vi "FlexMag - 24-03-2023.vi"() -> ()   [LabVIEW 2018] (continued)
        n3540 = local read "CH4_CC_DI"() -> (w5125:bool)
        n3541 = Compound Arithmetic op=OR(w5140, w5139, w5137, w5138) -> (w5141:bool)
        n3542 = case shown="False" w5131 {
          tunnel: [T13."Disabled and Grayed Out" ("Disabled") T13."Enabled" ("Disabled")] -> w5130
          frame False {
          }
          frame True {
          }
        }
        n3543 = case shown="False" w5132 {
          tunnel: [T13."Disabled and Grayed Out" ("Disabled") T13."Enabled" ("Disabled")] -> w5129
          frame False {
          }
          frame True {
          }
        }
        n3544 = case shown="False" w5141 {
          frame False {
            n3545 = local read "CH1_DS_DI"() -> (w5297:bool)
            n3546 = local read "CH2_DS_DI"() -> (w5296:bool)
            n3547 = local read "CH3_DS_DI"() -> (w5294:bool)
            n3548 = local read "CH4_DS_DI"() -> (w5295:bool)
            n3549 = Not(x=w5297) -> (.not. x?=w5298:bool)
            n3550 = Not(x=w5296) -> (.not. x?=w5293:bool)
            n3551 = Not(x=w5294) -> (.not. x?=w5292:bool)
            n3552 = Not(x=w5295) -> (.not. x?=w5291:bool)
            n3553 = property on="ch1_door_open" class="Str"("Visible"=w5298) -> ()  [unwired: 2 in, 2 out]
            n3554 = property on="ch2_door_open" class="Str"("Visible"=w5293) -> ()  [unwired: 2 in, 2 out]
            n3555 = property on="ch3_door_open" class="Str"("Visible"=w5292) -> ()  [unwired: 2 in, 2 out]
            n3556 = property on="ch4_door_open" class="Str"("Visible"=w5291) -> ()  [unwired: 2 in, 2 out]
          }
          frame True {
          }
        }
        n3557 = case shown="False" w5136 {
          tunnel: [T13."Disabled and Grayed Out" ("Disabled") T13."Enabled" ("Disabled")] -> w5135
          frame False {
          }
          frame True {
          }
        }
        n3558 = case shown="False" w5134 {
          tunnel: [T13."Disabled and Grayed Out" ("Disabled") T13."Enabled" ("Disabled")] -> w5133
          frame False {
          }
          frame True {
          }
        }
        n3559 = property on="ch1 cc mbar gui" class="DigNum (strict)"("Visible"=w5128) -> ()  [unwired: 2 in, 2 out]
        n3560 = property on="ch2 cc mbar gui" class="DigNum (strict)"("Visible"=w5127) -> ()  [unwired: 2 in, 2 out]
        n3561 = property on="ch3 cc mbar gui" class="DigNum (strict)"("Visible"=w5126) -> ()  [unwired: 2 in, 2 out]
        n3562 = property on="ch4 cc mbar gui" class="DigNum (strict)"("Visible"=w5125) -> ()  [unwired: 2 in, 2 out]
        n3563 = case shown="True" w5142 {
          frame False {
          }
          frame True {
            n3564 = local write "Warning Message"("Water Flow Problem !\nCheck Connections.." ("Warning Message")) -> ()
          }
        }
        n3565 = local write "Description"(w5164) -> ()
        n3566 = property on="Tp1 set speed gui" class="Bool"("DisabledEnum"=w5135) -> ()  [unwired: 2 in, 2 out]
        n3567 = property on="Tp1 normal speed gui" class="Bool"("DisabledEnum"=w5135) -> ()  [unwired: 2 in, 2 out]
        n3568 = property on="Tp1 low speed gui" class="Bool"("DisabledEnum"=w5135) -> ()  [unwired: 2 in, 2 out]
        n3569 = property on="Tp2 normal speed gui" class="Bool"("DisabledEnum"=w5133) -> ()  [unwired: 2 in, 2 out]
        n3570 = property on="Tp2 set speed gui" class="Bool"("DisabledEnum"=w5133) -> ()  [unwired: 2 in, 2 out]
        n3571 = property on="Tp2 low speed gui" class="Bool"("DisabledEnum"=w5133) -> ()  [unwired: 2 in, 2 out]
        n3572 = property on="Tp3 set speed gui" class="Bool"("DisabledEnum"=w5130) -> ()  [unwired: 2 in, 2 out]
        n3573 = property on="Tp3 normal speed gui" class="Bool"("DisabledEnum"=w5130) -> ()  [unwired: 2 in, 2 out]
        n3574 = property on="Tp3 low speed gui" class="Bool"("DisabledEnum"=w5130) -> ()  [unwired: 2 in, 2 out]
        n3575 = property on="Tp4 set speed gui" class="Bool"("DisabledEnum"=w5129) -> ()  [unwired: 2 in, 2 out]
        n3576 = property on="Tp4 normal speed gui" class="Bool"("DisabledEnum"=w5129) -> ()  [unwired: 2 in, 2 out]
        n3577 = property on="Tp4 low speed gui" class="Bool"("DisabledEnum"=w5129) -> ()  [unwired: 2 in, 2 out]
        n3578 = call <vilib>:"Draw Text at Point.vi"("[user-specified font]"=T12 {"Font Name:"="Bold", "Size"=20, "Strikeout?"=FALSE, "Italic?"=FALSE, "Underline?"=FALSE, "Outline?"=FALSE, "Shadow?"=FALSE, "Bold?"=TRUE}, "desired font(Application)"=T11."User-specified Font", "text"=w5163, "origin"=w5162, "picture"=w5165) -> ("new picture"=→"General View":picture)  [unwired: 5 in, 1 out]
      }
    }
    n3579 = Wait Until Next ms Multiple(millisecond multiple=u32 100) -> ()  [unwired: 1 out]
  }
  n3580 = property on="mp1 timer tab" class="TabCtl (strict)"("Visible"=w86) -> ()  [unwired: 2 in, 2 out]
  n3581 = property on="mp2 timer tab" class="TabCtl (strict)"("Visible"=w86) -> ()  [unwired: 2 in, 2 out]
  n3582 = property on="mp3 timer tab" class="TabCtl (strict)"("Visible"=w86) -> ()  [unwired: 2 in, 2 out]
  n3583 = property on="mp4 timer tab" class="TabCtl (strict)"("Visible"=w86) -> ()  [unwired: 2 in, 2 out]
  n3584 = property on="plvbv1 timer tab" class="TabCtl (strict)"("Visible"=w86) -> ()  [unwired: 2 in, 2 out]
  n3585 = property on="plvbv2 timer tab" class="TabCtl (strict)"("Visible"=w86) -> ()  [unwired: 2 in, 2 out]
  n3586 = property on="plvbv3 timer tab" class="TabCtl (strict)"("Visible"=w86) -> ()  [unwired: 2 in, 2 out]
  n3587 = property on="plvbv4 timer tab" class="TabCtl (strict)"("Visible"=w86) -> ()  [unwired: 2 in, 2 out]
  n3588 = property on="chvbv1 timer tab" class="TabCtl (strict)"("Visible"=w86) -> ()  [unwired: 2 in, 2 out]
  n3589 = property on="chvbv2 timer tab" class="TabCtl (strict)"("Visible"=w86) -> ()  [unwired: 2 in, 2 out]
  n3590 = property on="chvbv3 timer tab" class="TabCtl (strict)"("Visible"=w86) -> ()  [unwired: 2 in, 2 out]
  n3591 = property on="chvbv4 timer tab" class="TabCtl (strict)"("Visible"=w86) -> ()  [unwired: 2 in, 2 out]
  n3592 = property on="bgbv1 timer tab" class="TabCtl (strict)"("Visible"=w86) -> ()  [unwired: 2 in, 2 out]
  n3593 = property on="bgbv2 timer tab" class="TabCtl (strict)"("Visible"=w86) -> ()  [unwired: 2 in, 2 out]
  n3594 = property on="bgbv3 timer tab" class="TabCtl (strict)"("Visible"=w86) -> ()  [unwired: 2 in, 2 out]
  n3595 = property on="bgbv4 timer tab" class="TabCtl (strict)"("Visible"=w86) -> ()  [unwired: 2 in, 2 out]
  n3596 = property on="tpbv1 timer tab" class="TabCtl (strict)"("Visible"=w86) -> ()  [unwired: 2 in, 2 out]
  n3597 = property on="tpbv2 timer tab" class="TabCtl (strict)"("Visible"=w86) -> ()  [unwired: 2 in, 2 out]
  n3598 = property on="tpbv3 timer tab" class="TabCtl (strict)"("Visible"=w86) -> ()  [unwired: 2 in, 2 out]
  n3599 = property on="tpbv4 timer tab" class="TabCtl (strict)"("Visible"=w86) -> ()  [unwired: 2 in, 2 out]
  n3600 = property on="cc1 timer tab" class="TabCtl (strict)"("Visible"=w86) -> ()  [unwired: 2 in, 2 out]
  n3601 = property on="cc2 timer tab" class="TabCtl (strict)"("Visible"=w86) -> ()  [unwired: 2 in, 2 out]
  n3602 = property on="cc3 timer tab" class="TabCtl (strict)"("Visible"=w86) -> ()  [unwired: 2 in, 2 out]
  n3603 = property on="cc4 timer tab" class="TabCtl (strict)"("Visible"=w86) -> ()  [unwired: 2 in, 2 out]
  n3604 = property on="pcgv1 timer tab" class="TabCtl (strict)"("Visible"=w86) -> ()  [unwired: 2 in, 2 out]
  n3605 = property on="pcgv2 timer tab" class="TabCtl (strict)"("Visible"=w86) -> ()  [unwired: 2 in, 2 out]
  n3606 = property on="pcgv3 timer tab" class="TabCtl (strict)"("Visible"=w86) -> ()  [unwired: 2 in, 2 out]
  n3607 = property on="pcgv4 timer tab" class="TabCtl (strict)"("Visible"=w86) -> ()  [unwired: 2 in, 2 out]
  n3608 = property on="tp1 timer tab" class="TabCtl (strict)"("Visible"=w86) -> ()  [unwired: 2 in, 2 out]
  n3609 = property on="tp2 timer tab" class="TabCtl (strict)"("Visible"=w86) -> ()  [unwired: 2 in, 2 out]
  n3610 = property on="tp3 timer tab" class="TabCtl (strict)"("Visible"=w86) -> ()  [unwired: 2 in, 2 out]
  n3611 = property on="tp4 timer tab" class="TabCtl (strict)"("Visible"=w86) -> ()  [unwired: 2 in, 2 out]
  n3612 = property on="sov1 timer tab" class="TabCtl (strict)"("Visible"=w86) -> ()  [unwired: 2 in, 2 out]
  n3613 = property on="sov2 timer tab" class="TabCtl (strict)"("Visible"=w86) -> ()  [unwired: 2 in, 2 out]
  n3614 = property on="sov3 timer tab" class="TabCtl (strict)"("Visible"=w86) -> ()  [unwired: 2 in, 2 out]
  n3615 = property on="sov4 timer tab" class="TabCtl (strict)"("Visible"=w86) -> ()  [unwired: 2 in, 2 out]
  n3616 = property on="ch1 trnsbp left timer tab" class="TabCtl (strict)"("Visible"=w86) -> ()  [unwired: 2 in, 2 out]
  n3617 = property on="ch2 trnsbp right timer tab" class="TabCtl (strict)"("Visible"=w86) -> ()  [unwired: 2 in, 2 out]
  n3618 = property on="ch2 trnsbp left timer tab" class="TabCtl (strict)"("Visible"=w86) -> ()  [unwired: 2 in, 2 out]
  n3619 = property on="ch3 trnsbp right timer tab" class="TabCtl (strict)"("Visible"=w86) -> ()  [unwired: 2 in, 2 out]
  n3620 = property on="ch3 trnsbp left timer tab" class="TabCtl (strict)"("Visible"=w86) -> ()  [unwired: 2 in, 2 out]
  n3621 = property on="ch4 trnsbp right timer tab" class="TabCtl (strict)"("Visible"=w86) -> ()  [unwired: 2 in, 2 out]
  n3622 = property on="CH1-2 trnsgv timer tab" class="TabCtl (strict)"("Visible"=w86) -> ()  [unwired: 2 in, 2 out]
  n3623 = property on="CH2-3 trnsgv timer tab" class="TabCtl (strict)"("Visible"=w86) -> ()  [unwired: 2 in, 2 out]
  n3624 = property on="CH3-4 trnsgv timer tab" class="TabCtl (strict)"("Visible"=w86) -> ()  [unwired: 2 in, 2 out]
  n3625 = property on="ch1_door_open" class="Str"("Visible"=w30) -> ()  [unwired: 2 in, 2 out]
  n3626 = property on="ch2_door_open" class="Str"("Visible"=w30) -> ()  [unwired: 2 in, 2 out]
  n3627 = property on="ch3_door_open" class="Str"("Visible"=w30) -> ()  [unwired: 2 in, 2 out]
  n3628 = property on="ch4_door_open" class="Str"("Visible"=w30) -> ()  [unwired: 2 in, 2 out]
  n3629 = stacked-sequence {
    frame #0 {
      n3630 = Wait (ms)(milliseconds to wait=u32 100) -> ()  [unwired: 1 out]
      n3631 = flat-sequence {
        frame #0 {
          # "16 bit = 65536"
          # "MOXA 16 bit\n0-10V AI"
          n3632 = Divide(x=10.0, y=65536.0) -> (x/y=→"resolution":dbl)
        }
      }
      n3633 = property on="casette selection" class="Bool (strict)"("DisabledEnum"=T13."Disabled and Grayed Out" ("Disabled")) -> ()  [unwired: 2 in, 2 out]
      n3634 = local write "casette_ch1_gui"(FALSE) -> ()
      n3635 = local write "casette_ch2_gui"(FALSE) -> ()
      n3636 = local write "casette_ch3_gui"(FALSE) -> ()
      n3637 = local write "casette_ch4_gui"(FALSE) -> ()
      n3638 = local write "present location"(0.0 ("present location")) -> ()
    }
    frame #1 {
      n3639 = Wait (ms)(milliseconds to wait=u32 5000) -> ()  [unwired: 1 out]
    }
    frame #2 {
      n3640 = local read "CH3_Right_Limit_DI"() -> (w5527:bool)
      n3641 = local read "CH3_Right_Slow_DI"() -> (w5526:bool)
      n3642 = local read "CH1_Right_Limit_DI"() -> (w5533:bool)
      n3643 = local read "CH2_Right_Limit_DI"() -> (w5531:bool)
      n3644 = local read "CH1_Right_Slow_DI"() -> (w5532:bool)
      n3645 = local read "CH2_Right_Slow_DI"() -> (w5530:bool)
      n3646 = local read "CH3_Left_Limit_DI"() -> (w5525:bool)
      n3647 = local read "CH3_Left_Slow_DI"() -> (w5524:bool)
      n3648 = local read "CH2_Left_Limit_DI"() -> (w5529:bool)
      n3649 = local read "CH4_Left_Limit_DI"() -> (w5523:bool)
      n3650 = local read "CH2_Left_Slow_DI"() -> (w5528:bool)
      n3651 = local read "CH4_Left_Slow_DI"() -> (w5522:bool)
      n3652 = Compound Arithmetic op=OR(w5533, w5532) -> (w5521:bool)
      n3653 = Compound Arithmetic op=OR(w5531, w5530, w5529, w5528) -> (w5520:bool)
      n3654 = Compound Arithmetic op=OR(w5527, w5526, w5525, w5524) -> (w5519:bool)
      n3655 = Compound Arithmetic op=OR(w5523, w5522) -> (w5518:bool)
      n3656 = Build Array(FALSE ("element"), w5521, w5520, w5519, w5518) -> (w5535:bool[])
      n3657 = Boolean Array To Number(Boolean array=w5535) -> (number=w5537:u32)
      n3658 = Mantissa & Exponent(0:w5537) -> (2:w5536:dbl)  [unwired: 1 out]
      n3659 = case shown="1" w5536 {
        frame 0, Default {
        }
        frame 1 {
          n3660 = stacked-sequence {
            frame #0 {
              w5539 = u16 1 items=["CH1"=1, "CH2"=2, "CH3"=3, "CH4"=4] ("cassette position selection")
              n3661 = local write "cassette position selection"(w5539) -> ()
              n3662 = Wait (ms)(milliseconds to wait=u32 100) -> ()  [unwired: 1 out]
            }
            frame #1 {
              n3663 = local write "OK Button"(TRUE ("OK Button")) -> ()
            }
          }
        }
        frame 2 {
          n3664 = stacked-sequence {
            frame #0 {
              w5542 = u16 2 items=["CH1"=1, "CH2"=2, "CH3"=3, "CH4"=4] ("cassette position selection")
              n3665 = local write "cassette position selection"(w5542) -> ()
              n3666 = Wait (ms)(milliseconds to wait=u32 100) -> ()  [unwired: 1 out]
            }
            frame #1 {
              n3667 = local write "OK Button"(TRUE ("OK Button")) -> ()
            }
          }
        }
        frame 3 {
          n3668 = stacked-sequence {
            frame #0 {
              w5545 = u16 3 items=["CH1"=1, "CH2"=2, "CH3"=3, "CH4"=4] ("cassette position selection")
              n3669 = local write "cassette position selection"(w5545) -> ()
              n3670 = Wait (ms)(milliseconds to wait=u32 100) -> ()  [unwired: 1 out]
            }
            frame #1 {
              n3671 = local write "OK Button"(TRUE ("OK Button")) -> ()
            }
          }
        }
        frame 4 {
          n3672 = stacked-sequence {
            frame #0 {
              w5548 = u16 4 items=["CH1"=1, "CH2"=2, "CH3"=3, "CH4"=4] ("cassette position selection")
              n3673 = local write "cassette position selection"(w5548) -> ()
              n3674 = Wait (ms)(milliseconds to wait=u32 100) -> ()  [unwired: 1 out]
            }
            frame #1 {
              n3675 = local write "OK Button"(TRUE ("OK Button")) -> ()
            }
          }
        }
      }
    }
    frame #3 {
      # "cassette selection"
      n3676 = while {
        stop <- FALSE stop-if-true
        n3677 = Wait Until Next ms Multiple(millisecond multiple=u32 300) -> ()  [unwired: 1 out]
        n3678 = Equal?(x="service tab", y="IFWFLEXMAG") -> (x = y?=w5560:bool)
        n3679 = Equal?(x="ifwflexmag", y="service tab") -> (x = y?=w5561:bool)
        n3680 = case shown="True" "buzzer off" {
          frame False {
          }
          frame True {
            n3681 = local write "Buzzer DO"(FALSE ("Buzzer DO")) -> ()
          }
        }
        n3682 = case shown="True" "clear warning" {
          frame False {
          }
          frame True {
            n3683 = local write "Warning Message"("" ("Warning Message")) -> ()
          }
        }
        n3684 = case shown="True" "OK Button" {
          frame False {
          }
          frame True {
            n3685 = local write "OK Button"(FALSE ("OK Button")) -> ()
            n3686 = case shown="1" "cassette position selection" {
              frame 0, Default {
              }
              frame 1 {
                n3687 = local write "present location"(1.0 ("present location")) -> ()
                n3688 = local write "casette_ch1_gui"(TRUE) -> ()
                n3689 = local write "casette_ch2_gui"(FALSE) -> ()
                n3690 = local write "casette_ch3_gui"(FALSE) -> ()
                n3691 = local write "casette_ch4_gui"(FALSE) -> ()
              }
              frame 2 {
                n3692 = local write "present location"(2.0 ("present location")) -> ()
                n3693 = local write "casette_ch1_gui"(FALSE) -> ()
                n3694 = local write "casette_ch2_gui"(TRUE) -> ()
                n3695 = local write "casette_ch3_gui"(FALSE) -> ()
                n3696 = local write "casette_ch4_gui"(FALSE) -> ()
              }
              frame 3 {
                n3697 = local write "present location"(3.0 ("present location")) -> ()
                n3698 = local write "casette_ch1_gui"(FALSE) -> ()
                n3699 = local write "casette_ch2_gui"(FALSE) -> ()
                n3700 = local write "casette_ch3_gui"(TRUE) -> ()
                n3701 = local write "casette_ch4_gui"(FALSE) -> ()
              }
              frame 4 {
                n3702 = local write "present location"(4.0 ("present location")) -> ()
                n3703 = local write "casette_ch1_gui"(FALSE) -> ()
                n3704 = local write "casette_ch2_gui"(FALSE) -> ()
                n3705 = local write "casette_ch3_gui"(FALSE) -> ()
                n3706 = local write "casette_ch4_gui"(TRUE) -> ()
              }
            }
          }
        }
        n3707 = Or(x=w5561, y=w5560) -> (x .or. y?=w5559:bool)
        n3708 = And(x=w5559, y="show service tab") -> (x .and. y?=w5557:bool)
        n3709 = case shown="True" w5557 {
          frame False {
          }
          frame True {
            n3710 = property on="Technical Service" class="TabCtl (strict)"("Visible"=TRUE) -> ()  [unwired: 2 in, 2 out]
          }
        }
        n3711 = case shown="True" "hide service tab" {
          frame False {
          }
          frame True {
            n3712 = property on="Technical Service" class="TabCtl (strict)"("Visible"=FALSE) -> ()  [unwired: 2 in, 2 out]
            n3713 = local write "service tab"("" ("service tab")) -> ()
          }
        }
      }
      n3714 = flat-sequence {
        frame #0 {
          n3715 = Wait (ms)(milliseconds to wait=u32 100) -> ()  [unwired: 1 out]
          n3716 = property on="casette selection" class="Bool (strict)"("DisabledEnum"=T13."Enabled" ("Disabled")) -> ()  [unwired: 2 in, 2 out]
        }
      }
    }
  }
  n3717 = local write "ch1 desired pressure"(w88) -> ()
  n3718 = local write "ch2 desired pressure"(w88) -> ()
  n3719 = local write "ch3 desired pressure"(w88) -> ()
  n3720 = local write "ch4 desired pressure"(w88) -> ()
  n3721 = local write "water bypass"(FALSE ("water bypass")) -> ()
  n3722 = VISA Open(access mode=u32 0, VISA resource name="keysight port") -> (VISA resource name=w7:refnum<visa-resource-name>, error out=w8:errorcluster)  [unwired: 3 in]
  n3723 = call-poly "VISA Configure Serial Port"() -> ("error out"=w18:errorcluster)  [unwired: 9 in, 6 out]
  n3724 = VISA Clear(VISA resource name=w7, error in (no error)=w8) -> (VISA resource name out=w9:refnum<visa-resource-name>, error out=w10:errorcluster)
  n3725 = while {
    tunnel: "QR Scanner Com" -> [w5612]
    tunnel: w18 -> [w5613]
    tunnel: [w5611] -> w16
    tunnel: [w5601] -> w17
    stop <- FALSE stop-if-true
    n3726 = Or(x="QR continuous mode gui", y="QR continuous mode") -> (x .or. y?=w5594:bool)
    n3727 = Or(x="QR off mode", y="QR off mode gui") -> (x .or. y?=w5593:bool)
    n3728 = Wait Until Next ms Multiple(millisecond multiple=u32 300) -> ()  [unwired: 1 out]
    n3729 = Build Array(FALSE, "read", w5594, w5593, "QR reset", "QR save", "write") -> (w5609:bool[])
    n3730 = Boolean Array To Number(Boolean array=w5609) -> (number=w5610:u32)
    n3731 = Mantissa & Exponent(0:w5610) -> (2:w5608:dbl)  [unwired: 1 out]
    n3732 = case shown="0, Default" w5608 {
      tunnel: w5613 -> [w5620 w5639 w5669 w5691 w5716 w5741 w5762]
      tunnel: w5612 -> [w5621 w5638 w5668 w5690 w5715 w5740 w5761]
      tunnel: [w5619 w5637 w5666 w5688 w5713 w5738 w5759] -> w5611
      tunnel: [w5618 w5636 w5665 w5687 w5712 w5737 w5758] -> w5601
      tunnel: [w5617 "" ("read buffer") w5658 w5680 w5705 w5730 w5756] -> w5605
      tunnel: [w5622 TRUE w5659 w5681 w5706 w5731 w5757] -> w5604
      tunnel: [w5617 "" w5658 w5680 w5705 w5730 w5756] -> w5603
      frame 0, Default {
        n3733 = property class="Instr"(reference=w5621, error in=w5620) -> (reference out=w5626:refnum<visa-resource-name>, error out=w5625:errorcluster, "Serial Settings:Number of Bytes at Serial Port"=w5624:u32)
        n3734 = VISA Read(VISA resource name=w5626, byte count=w5624, error in (no error)=w5625) -> (VISA resource name out=w5619:refnum<visa-resource-name>, read buffer=w5617:string, error out=w5618:errorcluster)  [unwired: 1 out]
        "qr read statue" <- w5617
        n3735 = String Length(string=w5617) -> (length=w5623:i32)
        n3736 = Equal To 0?(x=w5623) -> (x = 0?=w5622:bool)
      }
      frame 1 {
        n3737 = Concatenate Strings("~\u0000", "\u0007", "\u0001", "\u0000\u0000", "\u0000") -> (w5631:string)
        n3738 = Concatenate Strings(w5631, "\u0011`") -> (w5632:string)
        n3739 = VISA Write(VISA resource name=w5638, write buffer=w5632, error in (no error)=w5639) -> (VISA resource name out=w5642:refnum<visa-resource-name>, error out=w5641:errorcluster)  [unwired: 1 out]
        n3740 = stacked-sequence {
          tunnel: [w5652] -> w5647
          tunnel: w5642 -> [w5652]
          tunnel: [w5651] -> w5646
          tunnel: w5641 -> [w5651]
          frame #0 {
            n3741 = Wait (ms)(milliseconds to wait=u32 40 ("millisecond multiple")) -> ()  [unwired: 1 out]
          }
        }
        n3742 = property class="Instr"(reference=w5647, error in=w5646) -> (reference out=w5645:refnum<visa-resource-name>, error out=w5644:errorcluster, "Serial Settings:Number of Bytes at Serial Port"=w5643:u32)
        n3743 = VISA Read(VISA resource name=w5645, byte count=w5643, error in (no error)=w5644) -> (VISA resource name out=w5637:refnum<visa-resource-name>, read buffer=→"read if asked":string, error out=w5636:errorcluster)  [unwired: 1 out]
      }
      frame 2 {
        (unwired) "ß\""
        (unwired) "Ö"
        (unwired) "ı"
        (unwired) "J+"
        n3744 = Concatenate Strings("~\u0000", "\b", "\u0001", "\u0000\u0000", "ê") -> (w5660:string)
        n3745 = Concatenate Strings(w5660, "(ı") -> (w5661:string)
        n3746 = VISA Write(VISA resource name=w5668, write buffer=w5661, error in (no error)=w5669) -> (VISA resource name out=w5655:refnum<visa-resource-name>, error out=w5654:errorcluster)  [unwired: 1 out]
        n3747 = stacked-sequence {
          tunnel: [w5678] -> w5657
          tunnel: w5655 -> [w5678]
          tunnel: [w5677] -> w5656
          tunnel: w5654 -> [w5677]
          frame #0 {
            n3748 = Wait (ms)(milliseconds to wait=u32 40 ("millisecond multiple")) -> ()  [unwired: 1 out]
          }
        }
        n3749 = local write "QR continuous mode"(FALSE ("QR continuous mode")) -> ()
        n3750 = property class="Instr"(reference=w5657, error in=w5656) -> (reference out=w5673:refnum<visa-resource-name>, error out=w5672:errorcluster, "Serial Settings:Number of Bytes at Serial Port"=w5671:u32)
        n3751 = VISA Read(VISA resource name=w5673, byte count=w5671, error in (no error)=w5672) -> (VISA resource name out=w5666:refnum<visa-resource-name>, read buffer=w5658:string, error out=w5665:errorcluster)  [unwired: 1 out]
        n3752 = String Length(string=w5658) -> (length=w5667:i32)
        n3753 = Equal To 0?(x=w5667) -> (x = 0?=w5659:bool)
      }
      frame 3 {
        n3754 = Concatenate Strings("~\u0000", "\b", "\u0001", "\u0000\u0000", "\u0000") -> (w5682:string)
        n3755 = Concatenate Strings(w5682, "t™") -> (w5683:string)
        n3756 = VISA Write(VISA resource name=w5690, write buffer=w5683, error in (no error)=w5691) -> (VISA resource name out=w5694:refnum<visa-resource-name>, error out=w5693:errorcluster)  [unwired: 1 out]
        n3757 = stacked-sequence {
          tunnel: [w5704] -> w5699
          tunnel: w5694 -> [w5704]
          tunnel: [w5703] -> w5698
          tunnel: w5693 -> [w5703]
          frame #0 {
            n3758 = Wait (ms)(milliseconds to wait=u32 40 ("millisecond multiple")) -> ()  [unwired: 1 out]
          }
        }
        n3759 = local write "QR off mode"(FALSE ("QR manual mode")) -> ()
        n3760 = property class="Instr"(reference=w5699, error in=w5698) -> (reference out=w5697:refnum<visa-resource-name>, error out=w5696:errorcluster, "Serial Settings:Number of Bytes at Serial Port"=w5695:u32)
        n3761 = VISA Read(VISA resource name=w5697, byte count=w5695, error in (no error)=w5696) -> (VISA resource name out=w5688:refnum<visa-resource-name>, read buffer=w5680:string, error out=w5687:errorcluster)  [unwired: 1 out]
        n3762 = String Length(string=w5680) -> (length=w5689:i32)
        n3763 = Equal To 0?(x=w5689) -> (x = 0?=w5681:bool)
      }
      frame 4 {
        n3764 = Concatenate Strings("~\u0000", "\t", "\u0001", "\u0000\u0000", "ÿ") -> (w5707:string)
        n3765 = Concatenate Strings(w5707, "À8") -> (w5708:string)
        n3766 = VISA Write(VISA resource name=w5715, write buffer=w5708, error in (no error)=w5716) -> (VISA resource name out=w5719:refnum<visa-resource-name>, error out=w5718:errorcluster)  [unwired: 1 out]
        n3767 = stacked-sequence {
          tunnel: [w5729] -> w5724
          tunnel: w5719 -> [w5729]
          tunnel: [w5728] -> w5723
          tunnel: w5718 -> [w5728]
          frame #0 {
            n3768 = Wait (ms)(milliseconds to wait=u32 40 ("millisecond multiple")) -> ()  [unwired: 1 out]
          }
        }
        n3769 = property class="Instr"(reference=w5724, error in=w5723) -> (reference out=w5722:refnum<visa-resource-name>, error out=w5721:errorcluster, "Serial Settings:Number of Bytes at Serial Port"=w5720:u32)
        n3770 = VISA Read(VISA resource name=w5722, byte count=w5720, error in (no error)=w5721) -> (VISA resource name out=w5713:refnum<visa-resource-name>, read buffer=w5705:string, error out=w5712:errorcluster)  [unwired: 1 out]
        n3771 = String Length(string=w5705) -> (length=w5714:i32)
        n3772 = Equal To 0?(x=w5714) -> (x = 0?=w5706:bool)
      }
      frame 5 {
        n3773 = Concatenate Strings("~\u0000", "\t", "\u0001", "\u0000\u0000", "\u0000") -> (w5732:string)
        n3774 = Concatenate Strings(w5732, "ŞÈ") -> (w5733:string)
        n3775 = VISA Write(VISA resource name=w5740, write buffer=w5733, error in (no error)=w5741) -> (VISA resource name out=w5744:refnum<visa-resource-name>, error out=w5743:errorcluster)  [unwired: 1 out]
        n3776 = stacked-sequence {
          tunnel: [w5754] -> w5749
          tunnel: w5744 -> [w5754]
          tunnel: [w5753] -> w5748
          tunnel: w5743 -> [w5753]
          frame #0 {
            n3777 = Wait (ms)(milliseconds to wait=u32 40 ("millisecond multiple")) -> ()  [unwired: 1 out]
          }
        }
        n3778 = property class="Instr"(reference=w5749, error in=w5748) -> (reference out=w5747:refnum<visa-resource-name>, error out=w5746:errorcluster, "Serial Settings:Number of Bytes at Serial Port"=w5745:u32)
        n3779 = VISA Read(VISA resource name=w5747, byte count=w5745, error in (no error)=w5746) -> (VISA resource name out=w5738:refnum<visa-resource-name>, read buffer=w5730:string, error out=w5737:errorcluster)  [unwired: 1 out]
        n3780 = String Length(string=w5730) -> (length=w5739:i32)
        n3781 = Equal To 0?(x=w5739) -> (x = 0?=w5731:bool)
      }
      frame 6 {
        n3782 = VISA Write(VISA resource name=w5761, write buffer="write buffer", error in (no error)=w5762) -> (VISA resource name out=w5764:refnum<visa-resource-name>, error out=w5763:errorcluster)  [unwired: 1 out]
        n3783 = stacked-sequence {
          tunnel: [w5772] -> w5769
          tunnel: w5764 -> [w5772]
          tunnel: [w5771] -> w5768
          tunnel: w5763 -> [w5771]
          frame #0 {
            n3784 = Wait (ms)(milliseconds to wait=u32 40 ("millisecond multiple")) -> ()  [unwired: 1 out]
          }
        }
        n3785 = property class="Instr"(reference=w5769, error in=w5768) -> (reference out=w5767:refnum<visa-resource-name>, error out=w5766:errorcluster, "Serial Settings:Number of Bytes at Serial Port"=w5765:u32)
        n3786 = VISA Read(VISA resource name=w5767, byte count=w5765, error in (no error)=w5766) -> (VISA resource name out=w5759:refnum<visa-resource-name>, read buffer=w5756:string, error out=w5758:errorcluster)  [unwired: 1 out]
        n3787 = String Length(string=w5756) -> (length=w5760:i32)
        n3788 = Equal To 0?(x=w5760) -> (x = 0?=w5757:bool)
      }
    }
    "error out 2" <- w5601
    "read buffer always" <- w5605
    n3789 = case shown="False" w5604 {
      tunnel: w5603 -> [w5616 _]
      frame False {
        "qr read buffer if available" <- w5616
      }
      frame True {
      }
    }
  }
  n3790 = while {
    tunnel: [w5781] -> w4
    tunnel: w9 -> [w5785]
    tunnel: w10 -> [w5784]
    tunnel: [w5782] -> w5
    stop <- FALSE stop-if-true
    n3791 = Build Array(FALSE, "case1") -> (w5788:bool[])
    n3792 = Boolean Array To Number(Boolean array=w5788) -> (number=w5789:u32)
    n3793 = Wait Until Next ms Multiple(millisecond multiple="keysight loop (ms)") -> ()  [unwired: 1 out]
    n3794 = Mantissa & Exponent(0:w5789) -> (2:w5787:dbl)  [unwired: 1 out]
    n3795 = case shown="0, Default" w5787 {
      tunnel: w5785 -> [w5797 w5817]
      tunnel: w5784 -> [w5796 w5816]
      tunnel: [w5802 w5822] -> w5783
      tunnel: [w5802 w5822] -> w5782
      tunnel: [w5801 w5821] -> w5781
      tunnel: "keysight wait time" -> [w5800 w5820]
      tunnel: [w5794 w5814] -> w5778
      frame 0, Default {
        n3796 = VISA Write(VISA resource name=w5797, write buffer="keysight default case", error in (no error)=w5796) -> (VISA resource name out=w5799:refnum<visa-resource-name>, error out=w5798:errorcluster)  [unwired: 1 out]
        n3797 = flat-sequence {
          tunnel: w5800 -> [w5810]
          tunnel: [w5809] -> w5806
          tunnel: w5799 -> [w5809]
          tunnel: w5798 -> [w5808]
          tunnel: [w5808] -> w5807
          frame #0 {
            n3798 = Wait (ms)(milliseconds to wait=w5810) -> ()  [unwired: 1 out]
          }
        }
        n3799 = VISA Read(VISA resource name=w5806, byte count=u32 256 ("Bytes at Port"), error in (no error)=w5807) -> (VISA resource name out=w5804:refnum<visa-resource-name>, read buffer=w5794:string, error out=w5803:errorcluster)  [unwired: 1 out]
        "read from keysight" <- w5794
        n3800 = flat-sequence {
          tunnel: w5800 -> [w5813]
          tunnel: [w5812] -> w5801
          tunnel: w5804 -> [w5812]
          tunnel: w5803 -> [w5811]
          tunnel: [w5811] -> w5802
          frame #0 {
            n3801 = Wait (ms)(milliseconds to wait=w5813) -> ()  [unwired: 1 out]
          }
        }
      }
      frame 1 {
        n3802 = VISA Write(VISA resource name=w5817, write buffer="keysight case 1", error in (no error)=w5816) -> (VISA resource name out=w5819:refnum<visa-resource-name>, error out=w5818:errorcluster)  [unwired: 1 out]
        n3803 = flat-sequence {
          tunnel: w5820 -> [w5830]
          tunnel: [w5829] -> w5826
          tunnel: w5819 -> [w5829]
          tunnel: w5818 -> [w5828]
          tunnel: [w5828] -> w5827
          frame #0 {
            n3804 = Wait (ms)(milliseconds to wait=w5830) -> ()  [unwired: 1 out]
          }
        }
        n3805 = VISA Read(VISA resource name=w5826, byte count=u32 256 ("Bytes at Port"), error in (no error)=w5827) -> (VISA resource name out=w5824:refnum<visa-resource-name>, read buffer=w5814:string, error out=w5823:errorcluster)  [unwired: 1 out]
        "read from keysight CASE 1" <- w5814
        n3806 = flat-sequence {
          tunnel: w5820 -> [w5833]
          tunnel: [w5832] -> w5821
          tunnel: w5824 -> [w5832]
          tunnel: w5823 -> [w5831]
          tunnel: [w5831] -> w5822
          frame #0 {
            n3807 = Wait (ms)(milliseconds to wait=w5833) -> ()  [unwired: 1 out]
          }
        }
      }
    }
    "error out keysight" <- w5783
    n3808 = Scan Value(string=w5778, format string="%f") -> (value=w5773:dbl)  [unwired: 1 in, 1 out]
    "keysight readout 2" <- w5773
    n3809 = Equal?(x=w5773, y=9.91e+37) -> (x = y?=w5774:bool)
    n3810 = case shown="True" w5774 {
      tunnel: [w5792 0.0 ("y")] -> w5777
      tunnel: w5773 -> [w5792 _]
      frame False {
      }
      frame True {
      }
    }
    "keysight readout" <- w5777
  }
  n3811 = disable-structure shown="Disabled" {
    disable-tunnel: "Microwave1 Com" -> [w5834 _]
    frame Disabled {
      w5835 = i16 1 items=["Unknown"=-1, "Unasserted"=0, "Asserted"=1] ("Serial Settings:Modem Line Settings:Line RTS State")
      w5836 = i16 0 items=["Unknown"=-1, "Unasserted"=0, "Asserted"=1] ("Serial Settings:Modem Line Settings:Line DTR State")
      n3812 = property class="Instr"(reference=w5834, "RTS State"=w5835) -> ()  [unwired: 1 in, 2 out]
      n3813 = property class="Instr"(reference=w5834, "DTR State"=w5836) -> ()  [unwired: 1 in, 2 out]
    }
    frame Enabled {
    }
  }
  n3814 = disable-structure shown="Disabled" {
    disable-tunnel: "Microwave2 Com" -> [w5837 _]
    frame Disabled {
      w5839 = i16 1 items=["Unknown"=-1, "Unasserted"=0, "Asserted"=1] ("Serial Settings:Modem Line Settings:Line RTS State")
      w5838 = i16 0 items=["Unknown"=-1, "Unasserted"=0, "Asserted"=1] ("Serial Settings:Modem Line Settings:Line DTR State")
      n3815 = property class="Instr"(reference=w5837, "RTS State"=w5839) -> ()  [unwired: 1 in, 2 out]
      n3816 = property class="Instr"(reference=w5837, "DTR State"=w5838) -> ()  [unwired: 1 in, 2 out]
    }
    frame Enabled {
    }
  }
  n3817 = call-poly "VISA Configure Serial Port"("VISA resource name"="Vat PC GV Com", "data bits (8)"=u16 7, "parity (0:none)"=enum16{"None", "Odd", "Even", "Mark", "Space"}."Even") -> ("VISA resource name out"=w96:refnum<visa-resource-name>, "error out"=w95:errorcluster)  [unwired: 11 in]
  n3818 = call "MB Serial Init.vi"("Baud Rate"=u32 115200, "VISA resource name"="TC2 Com") -> ("error out"=w81:errorcluster, "VISA resource name out"=w80:refnum<visa-resource-name>)  [unwired: 8 in]
  n3819 = call-poly "VISA Configure Serial Port"("VISA resource name"="RF Com", "timeout (10sec)"=u32 2000, "termination char\n(0xA = '\\n' = LF)"=u8 13 ("termination char\n(0xA = '\\n' = LF)"), "Enable Termination\nChar (T)"=TRUE ("Enable Termination\nChar (T)"), "baud rate (9600)"=u32 19200, "parity (0:none)"=enum16{"None", "Odd", "Even", "Mark", "Space"}."Odd") -> ("VISA resource name out"=w56:refnum<visa-resource-name>, "error out"=w57:errorcluster)  [unwired: 3 in, 5 out]
  n3820 = call-poly "VISA Configure Serial Port"("VISA resource name"="DCPS Com", "timeout (10sec)"=u32 2000, "termination char\n(0xA = '\\n' = LF)"=u8 13 ("termination char\n(0xA = '\\n' = LF)"), "Enable Termination\nChar (T)"=TRUE ("Enable Termination\nChar (T)"), "baud rate (9600)"=u32 19200, "parity (0:none)"=enum16{"None", "Odd", "Even", "Mark", "Space"}."Odd") -> ("VISA resource name out"=w65:refnum<visa-resource-name>, "error out"=w64:errorcluster)  [unwired: 3 in, 5 out]
  n3821 = call "MB Serial Init.vi"("Timeout"=u32 2000, "Mode"=enum16{"RTU", "ASCII"}."RTU", "Parity"=w146, "Baud Rate"=u32 9600, "VISA resource name"="Center I/O Com") -> ("error out"=w143:errorcluster, "VISA resource name out"=w144:refnum<visa-resource-name>)  [unwired: 5 in]
  n3822 = call-poly "VISA Configure Serial Port"("VISA resource name"="Microwave1 Com", "baud rate (9600)"="baud rate (9600) 1") -> ("VISA resource name out"=w27:refnum<visa-resource-name>, "error out"=w26:errorcluster)  [unwired: 12 in]
  n3823 = call "MB Serial Init.vi"("Timeout"=u32 2000, "Mode"=enum16{"RTU", "ASCII"}."RTU", "Parity"=w110, "Baud Rate"=u32 9600, "VISA resource name"="CH4 I/O Com") -> ("error out"=w112:errorcluster, "VISA resource name out"=w113:refnum<visa-resource-name>)  [unwired: 5 in]
  n3824 = call "MB Serial Init.vi"("Timeout"=u32 2000, "Mode"=enum16{"RTU", "ASCII"}."RTU", "Parity"=w117, "Baud Rate"=u32 9600, "VISA resource name"="CH3 I/O Com") -> ("error out"=w120:errorcluster, "VISA resource name out"=w119:refnum<visa-resource-name>)  [unwired: 5 in]
  n3825 = call "MB Serial Init.vi"("Timeout"=u32 2000, "Mode"=enum16{"RTU", "ASCII"}."RTU", "Parity"=w128, "Baud Rate"=u32 9600, "VISA resource name"="CH2 I/O Com") -> ("error out"=w125:errorcluster, "VISA resource name out"=w126:refnum<visa-resource-name>)  [unwired: 5 in]
  n3826 = call "MB Serial Init.vi"("Timeout"=u32 2000, "Mode"=enum16{"RTU", "ASCII"}."RTU", "Parity"=w37, "Baud Rate"=u32 9600, "VISA resource name"="Center I I/O Com") -> ("error out"=w34:errorcluster, "VISA resource name out"=w35:refnum<visa-resource-name>)  [unwired: 5 in]
  n3827 = call-poly "VISA Configure Serial Port"("VISA resource name"="Pfeiffer TP Com") -> ("VISA resource name out"=w94:refnum<visa-resource-name>, "error out"=w93:errorcluster)  [unwired: 6 in, 7 out]
  n3828 = call "MB Serial Init.vi"("Baud Rate"=u32 115200, "VISA resource name"="TC1 Com") -> ("error out"=w78:errorcluster, "VISA resource name out"=w77:refnum<visa-resource-name>)  [unwired: 8 in]
  n3829 = VISA Clear(VISA resource name=w65, error in (no error)=w64) -> (VISA resource name out=w70:refnum<visa-resource-name>, error out=w71:errorcluster)
  n3830 = VISA Clear(VISA resource name=w96, error in (no error)=w95) -> (VISA resource name out=w99:refnum<visa-resource-name>, error out=w100:errorcluster)
  n3831 = call "MB Serial Init.vi"("Timeout"=u32 2000, "Mode"=enum16{"RTU", "ASCII"}."RTU", "Parity"=w139, "Baud Rate"=u32 9600, "VISA resource name"="CH1 I/O Com") -> ("error out"=w134:errorcluster, "VISA resource name out"=w135:refnum<visa-resource-name>)  [unwired: 5 in]
  n3832 = VISA Clear(VISA resource name=w56, error in (no error)=w57) -> (VISA resource name out=w58:refnum<visa-resource-name>, error out=w59:errorcluster)
  n3833 = call-poly "VISA Configure Serial Port"("VISA resource name"="Microwave2 Com", "baud rate (9600)"="baud rate (9600) 2") -> ("VISA resource name out"=w24:refnum<visa-resource-name>, "error out"=w25:errorcluster)  [unwired: 12 in]
  n3834 = call "MB Serial Init.vi"("Timeout"=u32 2000, "Mode"=enum16{"RTU", "ASCII"}."RTU", "Parity"=w47, "Baud Rate"=u32 9600, "VISA resource name"="Counter Com") -> ("error out"=w44:errorcluster, "VISA resource name out"=w45:refnum<visa-resource-name>)  [unwired: 2 in, 3 out]
  n3835 = while {
    tunnel: w113 -> [w5846]
    tunnel: w112 -> [w5845]
    tunnel: [w5841] -> w106
    tunnel: [w5840] -> w105
    i -> [w5842]
    stop <- FALSE stop-if-true
    n3836 = Wait Until Next ms Multiple(millisecond multiple=u32 300) -> ()  [unwired: 1 out]
    n3837 = Less Or Equal?(x=w5842, y=5) -> (x <= y?=→"CH4 I/O Loading":bool)
    n3838 = stacked-sequence {
      seq-local: [w5851 _ _ _ _ _ _ _] -> [_ w5898 _ _ _ _ _ _]
      seq-local: [w5849 _ _ _ _ _ _ _] -> [_ w5896 _ _ _ _ _ _]
      seq-local: [_ w5897 _ _ _ _ _ _] -> [_ _ _ w5958 _ _ _ _]
      seq-local: [_ _ _ w5961 _ _ _ _] -> [_ _ _ _ w6009 _ _ _]
      seq-local: [_ _ _ _ w6007 _ _ _] -> [_ _ _ _ _ w6066 _ _]
      seq-local: [_ _ _ w5960 _ _ _ _] -> [_ _ _ _ w6006 _ _ _]
      seq-local: [_ w5895 _ _ _ _ _ _] -> [_ _ _ w5959 _ _ _ _]
      seq-local: [_ _ _ _ w6008 _ _ _] -> [_ _ _ _ _ w6067 _ _]
      tunnel: w5846 -> [w5852 _ _ _ _ _ _ _]
      tunnel: w5845 -> [w5850 _ _ _ _ _ _ _]
      tunnel: [_ _ _ _ _ w6063 _ _] -> w5841
      tunnel: [_ _ _ _ _ w6062 _ _] -> w5840
      frame #0 {
        # "CH4 DI 1&2"
        n3839 = call "MB Serial Master Query Read Discrete Inputs (poly).vi"("VISA resource name"=w5852, "Starting Address"=u16 0 ("Quantity"), "Quantity"=u16 8, "error in"=w5850, "Serial Parameters"=T15 {"Mode"=enum."RTU", "Slave Address"=1}) -> ("VISA resource name out"=w5885:refnum<visa-resource-name>, "Discrete Inputs"=w5869:bool[], "error out"=w5884:errorcluster)  [unwired: 11 in, 1 out]
        n3840 = Index Array(array=w5869, index #1=0 ("index"), index #2=1 ("index"), index #3=2 ("index"), index #4=3 ("index"), index #5=4 ("index"), index #6=5 ("index"), index #7=6 ("index"), index #8=7 ("index")) -> (element #1=→"CH4_MP_DI":bool, element #2=→"CH4_TP_BV_DI":bool, element #3=→"CH4_BG_BV_DI":bool, element #5=→"CH4_CH_ATM_DI":bool, element #7=→"CH4_PL_ATM_DI":bool, element #8=→"CH4_CC_DI":bool)  [unwired: 2 out]
        n3841 = call "MB Serial Master Query Read Discrete Inputs (poly).vi"("VISA resource name"=w5885, "Starting Address"=u16 0 ("Quantity"), "Quantity"=u16 8, "error in"=w5884, "Serial Parameters"=T15 {"Mode"=enum."RTU", "Slave Address"=2}) -> ("VISA resource name out"=w5851:refnum<visa-resource-name>, "Discrete Inputs"=w5853:bool[], "error out"=w5849:errorcluster)  [unwired: 11 in, 1 out]
        n3842 = Index Array(array=w5853, index #1=0 ("index"), index #2=1 ("index"), index #3=2 ("index"), index #4=3 ("index"), index #5=4 ("index"), index #6=5 ("index"), index #7=6 ("index"), index #8=7 ("index")) -> (element #2=→"CH4_M2_D2_DI":bool, element #3=→"CH4_M2_D3_DI":bool, element #4=→"CH4_Trns_BP_Right_DI":bool, element #5=→"CH4_Cst_Fix_Up_DI":bool, element #6=→"CH4_Cst_Fix_Down_DI":bool, element #7=→"CH4_PetCool_Up_DI":bool, element #8=→"CH4_PetCool_Down_DI":bool)  [unwired: 1 out]
      }
      frame #1 {
        # "CH4 DI 3&4"
        n3843 = call "MB Serial Master Query Read Discrete Inputs (poly).vi"("VISA resource name"=w5898, "Starting Address"=u16 0 ("Quantity"), "Quantity"=u16 8, "error in"=w5896, "Serial Parameters"=T15 {"Mode"=enum."RTU", "Slave Address"=3}) -> ("VISA resource name out"=w5933:refnum<visa-resource-name>, "Discrete Inputs"=w5916:bool[], "error out"=w5932:errorcluster)  [unwired: 11 in, 1 out]
        n3844 = Index Array(array=w5916, index #1=0 ("index"), index #2=1 ("index"), index #3=2 ("index"), index #4=3 ("index"), index #5=4 ("index"), index #6=5 ("index"), index #7=6 ("index"), index #8=7 ("index")) -> (element #1=→"CH4_SRV1_Piston_For_DI":bool, element #2=→"CH4_SRV1_Piston_Back_DI":bool, element #3=→"CH4_SRV_Start_Stop_DI":bool, element #4=→"CH4_SRV_Left_Direction_DI":bool, element #5=→"CH4_SRV2_COUNTER_DI":bool, element #6=→"CH4_M3_D6_DI":bool, element #7=w5892:bool, element #8=→"CH4_M3_D8_DI":bool)
        n3845 = local read "water bypass"() -> (w5894:bool)
        n3846 = case shown="True" w5894 {
          tunnel: w5892 -> [w5940 _]
          tunnel: [w5940 w5941] -> w5893
          frame False {
          }
          frame True {
            n3847 = local read "CH4_WFC_DO"() -> (w5941:bool)
          }
        }
        "CH4_WFC_DI" <- w5893
        n3848 = call "MB Serial Master Query Read Discrete Inputs (poly).vi"("VISA resource name"=w5933, "Starting Address"=u16 0 ("Quantity"), "Quantity"=u16 8, "error in"=w5932, "Serial Parameters"=T15 {"Mode"=enum."RTU", "Slave Address"=4}) -> ("VISA resource name out"=w5897:refnum<visa-resource-name>, "Discrete Inputs"=w5899:bool[], "error out"=w5895:errorcluster)  [unwired: 11 in, 1 out]
        n3849 = Index Array(array=w5899, index #1=0 ("index"), index #2=1 ("index"), index #3=2 ("index"), index #4=3 ("index"), index #5=4 ("index"), index #6=5 ("index"), index #7=6 ("index"), index #8=7 ("index")) -> (element #1=→"CH4_Air_Pressure_DI":bool, element #2=→"CH4_DS_DI":bool, element #3=→"CH4_TGV_Control_DI":bool, element #4=→"CH4_Trns_Interlock_DI":bool, element #5=→"CH4_M4_D5_DI":bool, element #6=→"CH4_M4_D6_DI":bool, element #7=→"CH4_Left_Slow_DI":bool, element #8=→"CH4_Left_Limit_DI":bool)
      }
      frame #2 {
        n3850 = local read "CH4 I/O Loading"() -> (w5942:bool)
        n3851 = case shown="True" w5942 {
          frame False {
          }
          frame True {
            n3852 = local read "CH4_SRV1_Piston_Back_DI"() -> (w5953:bool)
            n3853 = local read "CH4_SRV1_Piston_For_DI"() -> (w5952:bool)
            n3854 = local read "CH4_BG_BV_DI"() -> (w5950:bool)
            n3855 = local read "CH4_TP_BV_DI"() -> (w5949:bool)
            n3856 = local read "CH4_MP_DI"() -> (w5948:bool)
            n3857 = local read "CH4_WFC_DI"() -> (w5954:bool)
            n3858 = local read "CH4_CC_DI"() -> (w5951:bool)
            n3859 = local write "CH4_MP_DO"(w5948) -> ()
            n3860 = local write "CH4_TP_BV_DO"(w5949) -> ()
            n3861 = local write "CH4_BG_BV_DO"(w5950) -> ()
            n3862 = local write "CH4_CC_DO"(w5951) -> ()
            n3863 = local write "CH4_SRV1_Piston_For_DO"(w5952) -> ()
            n3864 = local write "CH4_SRV1_Piston_Back_DO"(w5953) -> ()
            n3865 = local write "CH4_WFC_DO"(w5954) -> ()
            n3866 = local read "CH4_PetCool_Down_DI"() -> (w5944:bool)
            n3867 = local read "CH4_Cst_Fix_Down_DI"() -> (w5947:bool)
            n3868 = local read "CH4_Trns_BP_Right_DI"() -> (w5946:bool)
            n3869 = local read "CH4_PetCool_Up_DI"() -> (w5945:bool)
            n3870 = local read "CH4_TGV_Control_DI"() -> (w5943:bool)
            n3871 = local write "CH4_Trns_BP_Right_DO"(w5946) -> ()
            n3872 = local write "CH4_Cst_Fix_DO"(w5947) -> ()
            n3873 = local write "CH4_PetCool_Up_DO"(w5945) -> ()
            n3874 = local write "CH4_PetCool_Down_DO"(w5944) -> ()
            n3875 = local write "CH4_TGV_Control_DO"(w5943) -> ()
          }
        }
      }
      frame #3 {
        # "CH4 DO 1&2"
        n3876 = local read "CH4 I/O Loading"() -> (w5962:bool)
        n3877 = case shown="False" w5962 {
          tunnel: [w5974 w5983] -> w5964
          tunnel: ["CH4_PL_VBV_DO" w5981] -> w5957
          tunnel: ["CH4_CH_VBV_DO" w5981] -> w5956
          frame False {
            n3878 = Build Array("CH4_MP_DO", "CH4_TP_BV_DO", "CH4_BG_BV_DO", "CH4_CH_VBV_DO", "CH4_CH_ATM_DO", "CH4_PL_VBV_DO", "CH4_PL_ATM_DO", "CH4_CC_DO") -> (w5974:bool[])
          }
          frame True {
            w5981 = FALSE
            w5982 = FALSE
            n3879 = local read "CH4_BG_BV_DI"() -> (w5986:bool)
            n3880 = local read "CH4_TP_BV_DI"() -> (w5985:bool)
            n3881 = local read "CH4_MP_DI"() -> (w5984:bool)
            n3882 = local read "CH4_CC_DI"() -> (w5987:bool)
            n3883 = Build Array(w5984, w5985, w5986, w5982, w5982, w5982, w5981, w5987) -> (w5983:bool[])
          }
        }
        "CH4_CH_VBV_DI" <- w5956
        "CH4_PL_VBV_DI" <- w5957
        n3884 = call "MB Serial Master Query Write Multiple Coils (poly).vi"("VISA resource name"=w5958, "Starting Address"=u16 320, "Coils"=w5964, "error in"=w5959, "Serial Parameters"=T15 {"Mode"=enum."RTU", "Slave Address"=1}) -> ("VISA resource name out"=w5967:refnum<visa-resource-name>, "error out"=w5966:errorcluster)  [unwired: 12 in, 1 out]
        n3885 = local read "CH4 I/O Loading"() -> (w5963:bool)
        n3886 = case shown="False" w5963 {
          tunnel: [w5989 w6005] -> w5965
          tunnel: ["CH4_SoV_Ar_DO" w5997] -> w5955
          frame False {
            n3887 = Build Array("CH4_SoV_Ar_DO", "CH4_M2_D2_DO", "CH4_M2_D3_DO", "CH4_Trns_BP_Right_DO", "CH4_Cst_Fix_DO", "CH4_M2_D6_DO", "CH4_PetCool_Up_DO", "CH4_PetCool_Down_DO") -> (w5989:bool[])
          }
          frame True {
            w5997 = FALSE
            n3888 = local read "CH4_PetCool_Down_DI"() -> (w5998:bool)
            n3889 = local read "CH4_Trns_BP_Right_DI"() -> (w6002:bool)
            n3890 = local read "CH4_Cst_Fix_Down_DI"() -> (w6001:bool)
            n3891 = local read "CH4_PetCool_Up_DI"() -> (w5999:bool)
            n3892 = local read "CH4_M2_D2_DI"() -> (w6004:bool)
            n3893 = local read "CH4_M2_D3_DI"() -> (w6003:bool)
            n3894 = Build Array(w5997, w6004, w6003, w6002, w6001, FALSE ("element"), w5999, w5998) -> (w6005:bool[])
          }
        }
        "CH4_SoV_Ar_DI" <- w5955
        n3895 = call "MB Serial Master Query Write Multiple Coils (poly).vi"("VISA resource name"=w5967, "Starting Address"=u16 320, "Coils"=w5965, "error in"=w5966, "Serial Parameters"=T15 {"Mode"=enum."RTU", "Slave Address"=2}) -> ("VISA resource name out"=w5961:refnum<visa-resource-name>, "error out"=w5960:errorcluster)  [unwired: 12 in, 1 out]
      }
      frame #4 {
        # "CH4 DO 3&4"
        n3896 = local read "CH4 I/O Loading"() -> (w6012:bool)
        n3897 = case shown="False" w6012 {
          tunnel: [w6033 w6043] -> w6013
          frame False {
            n3898 = Build Array("CH4_SRV1_Piston_For_DO", "CH4_SRV1_Piston_Back_DO", "CH4_M3_D3_DO", "CH4_SRV_Direction_Clockwise_DO", "CH4_M3_D5_DO", "CH4_M3_D6_DO", "CH4_WFC_DO", "CH4_M3_D8_DO") -> (w6033:bool[])
          }
          frame True {
            w6042 = FALSE
            n3899 = local read "CH4_SRV1_Piston_Back_DI"() -> (w6045:bool)
            n3900 = local read "CH4_SRV1_Piston_For_DI"() -> (w6044:bool)
            n3901 = local read "CH4_M3_D8_DI"() -> (w6048:bool)
            n3902 = local read "CH4_M3_D6_DI"() -> (w6046:bool)
            n3903 = local read "CH4_WFC_DI"() -> (w6047:bool)
            n3904 = Build Array(w6044, w6045, w6042, w6042, w6042, w6046, w6047, w6048) -> (w6043:bool[])
          }
        }
        n3905 = call "MB Serial Master Query Write Multiple Coils (poly).vi"("VISA resource name"=w6009, "Starting Address"=u16 320, "Coils"=w6013, "error in"=w6006, "Serial Parameters"=T15 {"Mode"=enum."RTU", "Slave Address"=3}) -> ("VISA resource name out"=w6015:refnum<visa-resource-name>, "error out"=w6014:errorcluster)  [unwired: 12 in, 1 out]
        n3906 = local read "CH4 I/O Loading"() -> (w6011:bool)
        n3907 = case shown="False" w6011 {
          tunnel: [w6020 w6030] -> w6010
          frame False {
            n3908 = Build Array("CH4_LN2_DO", "CH4_M4_D2_DO", "CH4_TGV_Control_DO", "CH4_M4_D4_DO", "CH4_M4_D5_DO", "CH4_M4_D6_DO", "CH4_Left_Slow_DO", "CH4_Left_Limit_DO") -> (w6020:bool[])
          }
          frame True {
            w6031 = FALSE
            w6032 = FALSE
            n3909 = local read "CH4_TGV_Control_DI"() -> (w6029:bool)
            n3910 = Build Array(w6032, w6032, w6029, w6031, w6031, w6031, w6031, w6031) -> (w6030:bool[])
          }
        }
        n3911 = call "MB Serial Master Query Write Multiple Coils (poly).vi"("VISA resource name"=w6015, "Starting Address"=u16 320, "Coils"=w6010, "error in"=w6014, "Serial Parameters"=T15 {"Mode"=enum."RTU", "Slave Address"=4}) -> ("VISA resource name out"=w6008:refnum<visa-resource-name>, "error out"=w6007:errorcluster)  [unwired: 12 in, 1 out]
      }
      frame #5 {
        # "CH4 AI&AO"
        n3912 = call "MB Serial Master Query Read Input Registers (poly).vi"("VISA resource name"=w6067, "Starting Address"=u16 704, "Quantity"=u16 8, "error in"=w6066, "Serial Parameters"=T15 {"Mode"=enum."RTU", "Slave Address"=5}) -> ("VISA resource name out"=w6065:refnum<visa-resource-name>, "Input Registers"=w6078:u16[], "error out"=w6064:errorcluster)  [unwired: 11 in, 1 out]
        n3913 = Index Array(array=w6078, index #1=0 ("index"), index #2=1 ("index"), index #3=2 ("index"), index #4=3 ("index"), index #5=4 ("index"), index #6=5 ("index"), index #7=6 ("index"), index #8=7 ("index")) -> (element #1=→"CH4_Ai_Pl_Pg":u16, element #2=→"CH4_Ai_Ch_Pg":u16, element #3=→"CH4_Ai_Ch_Cc":u16, element #4=→"CH4_Ai_A4":u16, element #5=→"CH4_Ai_A5":u16, element #6=→"CH4_Ai_A6":u16, element #7=→"CH4_LN2_TK_t":u16, element #8=→"CH4_LN2_TK_b":u16)
        n3914 = Build Array(FALSE, "CH4 AO1 Set", "CH4 AO2 Set", "CH4 AO3 Set", "CH4 AO4 Set") -> (w6058:bool[])
        n3915 = Boolean Array To Number(Boolean array=w6058) -> (number=w6059:u32)
        n3916 = Mantissa & Exponent(0:w6059) -> (2:w6052:dbl)  [unwired: 1 out]
        n3917 = case shown="1" w6052 {
          tunnel: [0.0 ("TC2_Set_Value") "CH4 AO1" "CH4 AO2" "CH4 AO3" "CH4 AO4"] -> w6051
          tunnel: [0 1184 1185 1186 1187] -> w6049
          frame 0, Default {
          }
          frame 1 {
            n3918 = local write "CH4 AO1 Set"(FALSE ("CH1 AO1 Set")) -> ()
          }
          frame 2 {
            n3919 = local write "CH4 AO2 Set"(FALSE ("CH1 AO2 Set")) -> ()
          }
          frame 3 {
            n3920 = local write "CH4 AO3 Set"(FALSE ("CH1 AO3 Set")) -> ()
          }
          frame 4 {
            n3921 = local write "CH4 AO4 Set"(FALSE ("CH2 AO4 Set")) -> ()
          }
        }
        n3922 = Build Array(w6051) -> (w6050:dbl[])
        n3923 = call "MB Serial Master Query Write Multiple Registers (poly).vi"("VISA resource name"=w6065, "Starting Address"=w6049, "Registers"=w6050, "error in"=w6064, "Serial Parameters"=T15 {"Mode"=enum."RTU", "Slave Address"=6}) -> ("VISA resource name out"=w6063:refnum<visa-resource-name>, "error out"=w6062:errorcluster)  [unwired: 12 in, 1 out]
      }
      frame #6 {
      }
      frame #7 {
      }
    }
  }
  n3924 = while {
    tunnel: w135 -> [w6107]
    tunnel: w134 -> [w6106]
    tunnel: [w6102] -> w132
    tunnel: [w6101] -> w133
    i -> [w6103]
    stop <- FALSE stop-if-true
    n3925 = Wait Until Next ms Multiple(millisecond multiple=u32 300) -> ()  [unwired: 1 out]
    n3926 = Less Or Equal?(x=w6103, y=5) -> (x <= y?=→"CH1 I/O Loading":bool)
    n3927 = stacked-sequence {
      seq-local: [w6111 _ _ _ _ _ _ _] -> [_ w6159 _ _ _ _ _ _]
      seq-local: [w6110 _ _ _ _ _ _ _] -> [_ w6158 _ _ _ _ _ _]
      seq-local: [_ w6156 _ _ _ _ _ _] -> [_ _ _ w6224 _ _ _ _]
      seq-local: [_ w6157 _ _ _ _ _ _] -> [_ _ _ w6223 _ _ _ _]
      seq-local: [_ _ _ w6221 _ _ _ _] -> [_ _ _ _ w6272 _ _ _]
      seq-local: [_ _ _ w6222 _ _ _ _] -> [_ _ _ _ w6271 _ _ _]
      seq-local: [_ _ _ _ w6269 _ _ _] -> [_ _ _ _ _ w6345 _ _]
      seq-local: [_ _ _ _ w6270 _ _ _] -> [_ _ _ _ _ w6342 _ _]
      tunnel: w6107 -> [w6113 _ _ _ _ _ _ _]
      tunnel: w6106 -> [w6112 _ _ _ _ _ _ _]
      tunnel: [_ _ _ _ _ w6348 _ _] -> w6102
      tunnel: [_ _ _ _ _ w6347 _ _] -> w6101
      frame #0 {
        # "CH1 DI 1&2"
        n3928 = call "MB Serial Master Query Read Discrete Inputs (poly).vi"("VISA resource name"=w6113, "Starting Address"=u16 0 ("Quantity"), "Quantity"=u16 8, "error in"=w6112, "Serial Parameters"=T15 {"Mode"=enum."RTU", "Slave Address"=1}) -> ("VISA resource name out"=w6131:refnum<visa-resource-name>, "Discrete Inputs"=w6135:bool[], "error out"=w6130:errorcluster)  [unwired: 11 in, 1 out]
        n3929 = Index Array(array=w6135, index #1=0 ("index"), index #2=1 ("index"), index #3=2 ("index"), index #4=3 ("index"), index #5=4 ("index"), index #6=5 ("index"), index #7=6 ("index"), index #8=7 ("index")) -> (element #1=→"CH1_MP_DI":bool, element #2=→"CH1_TP_BV_DI":bool, element #3=→"CH1_BG_BV_DI":bool, element #5=→"CH1_CH_ATM_DI":bool, element #7=→"CH1_PL_ATM_DI":bool, element #8=→"CH1_CC_DI":bool)  [unwired: 2 out]
        n3930 = call "MB Serial Master Query Read Discrete Inputs (poly).vi"("VISA resource name"=w6131, "Starting Address"=u16 0 ("Quantity"), "Quantity"=u16 8, "error in"=w6130, "Serial Parameters"=T15 {"Mode"=enum."RTU", "Slave Address"=2}) -> ("VISA resource name out"=w6111:refnum<visa-resource-name>, "Discrete Inputs"=w6114:bool[], "error out"=w6110:errorcluster)  [unwired: 11 in, 1 out]
        n3931 = Index Array(array=w6114, index #1=0 ("index"), index #2=1 ("index"), index #3=2 ("index"), index #4=3 ("index"), index #5=4 ("index"), index #6=5 ("index"), index #7=6 ("index"), index #8=7 ("index")) -> (element #2=→"CH1_Trns_Gv_Open_DI":bool, element #3=→"CH1_Trns_Gv_Close_DI":bool, element #4=→"CH1_M2_D4_DI":bool, element #5=→"CH1_Cst_Fix_Up_DI":bool, element #6=→"CH1_Cst_Fix_Down_DI":bool, element #7=→"CH1_PetCool_Up_DI":bool, element #8=→"CH1_PetCool_Down_DI":bool)  [unwired: 1 out]
      }
      frame #1 {
        # "CH1 DI 3&4"
        n3932 = call "MB Serial Master Query Read Discrete Inputs (poly).vi"("VISA resource name"=w6159, "Starting Address"=u16 0 ("Quantity"), "Quantity"=u16 8, "error in"=w6158, "Serial Parameters"=T15 {"Mode"=enum."RTU", "Slave Address"=3}) -> ("VISA resource name out"=w6194:refnum<visa-resource-name>, "Discrete Inputs"=w6177:bool[], "error out"=w6193:errorcluster)  [unwired: 11 in, 1 out]
        n3933 = Index Array(array=w6177, index #1=0 ("index"), index #2=1 ("index"), index #3=2 ("index"), index #4=3 ("index"), index #5=4 ("index"), index #6=5 ("index"), index #7=6 ("index"), index #8=7 ("index")) -> (element #1=→"CH1_SRV1_Piston_For_DI":bool, element #2=→"CH1_SRV1_Piston_Back_DI":bool, element #3=→"CH1_SRV_Start_Stop_DI":bool, element #4=→"CH1_SRV_Left_Direction_DI":bool, element #5=→"CH1_SRV2_COUNTER_DI":bool, element #6=→"CH1_M3_D6_DI":bool, element #7=w6154:bool, element #8=→"CH1_Trns_BP_Left_DI":bool)
        n3934 = local read "water bypass"() -> (w6155:bool)
        n3935 = case shown="True" w6155 {
          tunnel: w6154 -> [w6201 _]
          tunnel: [w6201 w6202] -> w6153
          frame False {
          }
          frame True {
            n3936 = local read "CH1_WFC_DO"() -> (w6202:bool)
          }
        }
        "CH1_WFC_DI" <- w6153
        n3937 = call "MB Serial Master Query Read Discrete Inputs (poly).vi"("VISA resource name"=w6194, "Starting Address"=u16 0 ("Quantity"), "Quantity"=u16 8, "error in"=w6193, "Serial Parameters"=T15 {"Mode"=enum."RTU", "Slave Address"=4}) -> ("VISA resource name out"=w6156:refnum<visa-resource-name>, "Discrete Inputs"=w6160:bool[], "error out"=w6157:errorcluster)  [unwired: 11 in, 1 out]
        n3938 = Index Array(array=w6160, index #1=0 ("index"), index #2=1 ("index"), index #3=2 ("index"), index #4=3 ("index"), index #5=4 ("index"), index #6=5 ("index"), index #7=6 ("index"), index #8=7 ("index")) -> (element #1=→"CH1_Air_Pressure_DI":bool, element #2=→"CH1_DS_DI":bool, element #3=→"CH1_TGV_Control_DI":bool, element #4=→"CH1_Trns_Interlock_DI":bool, element #5=→"CH1_Right_Limit_DI":bool, element #6=→"CH1_Right_Slow_DI":bool, element #7=→"CH1_M4_D7_DI":bool, element #8=→"CH1_M4_D8_DI":bool)
      }
      frame #2 {
        n3939 = local read "CH1 I/O Loading"() -> (w6203:bool)
        n3940 = case shown="True" w6203 {
          frame False {
          }
          frame True {
            n3941 = local read "CH1_SRV1_Piston_Back_DI"() -> (w6215:bool)
            n3942 = local read "CH1_BG_BV_DI"() -> (w6206:bool)
            n3943 = local read "CH1_SRV1_Piston_For_DI"() -> (w6216:bool)
            n3944 = local read "CH1_TP_BV_DI"() -> (w6207:bool)
            n3945 = local read "CH1_MP_DI"() -> (w6204:bool)
            n3946 = local read "CH1_CC_DI"() -> (w6205:bool)
            n3947 = local read "CH1_Trns_BP_Left_DI"() -> (w6213:bool)
            n3948 = local read "CH1_WFC_DI"() -> (w6214:bool)